vi "USRP(receiver,9600).vi"() -> ()   [LabVIEW 2013]
uses:
  <vilib>/Analysis/2dsp.llb/Complex FFT.vi
  <vilib>/Analysis/2dsp.llb/Inverse Complex FFT.vi
  Combination device(9600).vi
  common/path deletes.vi
  common/Viterbi.vi
  FER(9600).vi
  common/metrics.vi
  transmitter/9600/syndrom(9600).vi
  <instrlib>/niUSRP/niUSRP Fetch Rx Data (CDB).vi
  Gateway(9600).vi
  <vilib>/Analysis/NI_AALPro.lvlib
  <vilib>/ptbypt/NI_PtbyPt.lvlib
panel:
  in  "Номер\nканала":i32
  in  "IQ rate":dbl=850000.0 format="%#_13g"
  in  "gain":dbl format="%#_6f"
  in  "device name":refnum<k15>="192.168.10.2"
  in  "freq.":dbl=850000000.0 format="%#_6p"
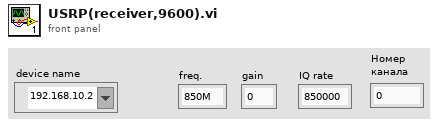
[diagram p1: front panel]
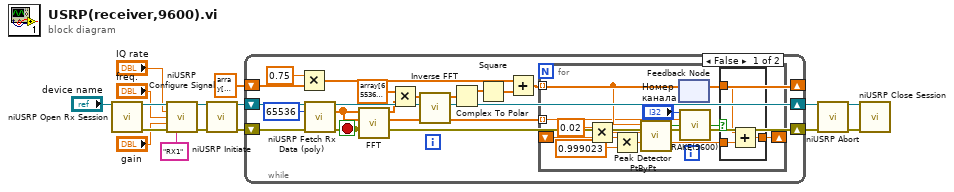
[diagram p0: block diagram]
diagram:
  n1 = call <instrlib>:"niUSRP Open Rx Session.vi"("device names"="device name") -> ("session handle out"=w16:refnum<k15>, "error out"=w15:errorcluster)  [unwired: 13 in]
  n2 = call <instrlib>:"niUSRP Configure Signal.vi"("session handle"=w16, "IQ rate"="IQ rate", "carrier frequency"="freq.", "gain"="gain", "error in (no error)"=w15, "active antenna"="RX1") -> ("session handle out"=w9:refnum<k15>, "error out"=w8:errorcluster)  [unwired: 5 in, 3 out]
  n3 = call <instrlib>:"niUSRP Initiate.vi"("session handle"=w9, "error in (no error)"=w8) -> ("session handle out"=w7:refnum<k15>, "error out"=w6:errorcluster)  [unwired: 12 in]
  n4 = while {
    shift-right: [w31] -> w4
    shift-left: w6 -> [w32]
    shift-right: [w28] -> w2
    shift-left: w7 -> [w29]
    shift-right: [w22] -> _
    shift-left: dbl[] array[65536 elements] -> [w19]
    stop <- w31 stop-if-true
    n5 = Multiply(x=0.75, y=w19) -> (x*y=w20:dbl[])
    n6 = call-poly <instrlib>:"niUSRP Fetch Rx Data (poly).vi"("session handle"=w29, "number of samples"=65536 ("channel 2"), "error in (no error)"=w32) -> ("session handle out"=w28:refnum<k15>, "data"=w21:cdb[], "error out"=w31:errorcluster)  [unwired: 9 in, 1 out]
    n7 = call-poly <vilib>:"FFT.vi"("X"=w21) -> ("FFT {X}"=w27:cdb[])  [unwired: 9 in, 1 out]
    n8 = Multiply(x=cdb[] array[65536 elements] ("for path searcher"), y=w27) -> (x*y=w30:cdb[])
    n9 = call-poly <vilib>:"Inverse FFT.vi"("FFT {X}"=w30) -> ("X"=w25:cdb[])  [unwired: 9 in, 1 out]
    n10 = Complex To Polar(r * e^(i*theta)=w25) -> (r=w24:dbl[])  [unwired: 1 out]
    n11 = Square(x=w24) -> (x^2=w23:dbl[])
    n12 = Add(x=w20, y=w23) -> (x+y=w22:dbl[])
    n13 = for {
      shift-right: [w36] -> _
      shift-left: _ -> [w41]
      tunnel: w22 -> [w35] mode=indexing
      tunnel: w21 -> [w33] mode=indexing
      n14 = Multiply(x=0.02 ("y"), y=w41) -> (x*y=w43:dbl)
      n15 = Multiply(x=w41, y=0.999023) -> (x*y=w37:dbl)
      n16 = call <vilib>:"Peak Detector PtByPt.vi"("x"=w35, "threshold peak"=w43) -> ("peak"=w38:bool)  [unwired: 3 in, 2 out]
      n17 = feedback #1() -> (w34:dbl)  [unwired: 1 in]
      n18 = feedback-in #1(w35) -> ()
      n19 = call "RAKE(9600).vi"("Номер\nканала"="Номер\nканала", "ВЫБОРКА"=w33, "add"=w38) -> ()  [unwired: 13 in]
      n20 = case shown="False" w38 {
        tunnel: w37 -> [w46 w47]
        tunnel: [w45 w47] -> w36
        tunnel: w34 -> [w44 _]
        frame False {
          n21 = Add(x=w44, y=w46) -> (x+y=w45:dbl)
        }
        frame True {
        }
      }
    }
  }
  n22 = call <instrlib>:"niUSRP Abort.vi"("session handle"=w2, "error in (no error)"=w4) -> ("session handle out"=w5:refnum<k15>, "error out"=w3:errorcluster)  [unwired: 12 in]
  n23 = call <instrlib>:"niUSRP Close Session.vi"("session handle"=w5, "error in (no error)"=w3) -> ()  [unwired: 13 in, 1 out]
